vi "Dresden R2R Sputter 03.02.2018 IY24.vi"() -> ()   [LabVIEW 2009] (continued)
                                }
                                frame #4 {
                                n27061 = Wait (ms)(milliseconds to wait=u32 100) -> ()  [unwired: 1 out]
                                n27062 = local write "Parameters_auto_set"(TRUE ("Parameters_auto_set")) -> ()
                                }
                                frame #5 {
                                n27063 = while {
                                i -> [w32211]
                                stop <- w32207 stop-if-true
                                n27064 = Wait Until Next ms Multiple(millisecond multiple=u32 300) -> ()  [unwired: 1 out]
                                n27065 = Greater?(x=w32211, y=100) -> (0:w32208:bool)
                                n27066 = local read "Parameters_auto_set"() -> (w32212:bool)
                                n27067 = case shown="False" w32212 {
                                tunnel: [TRUE FALSE] -> w32209
                                frame #0 {
                                }
                                frame #1 {
                                }
                                }
                                n27068 = Or(x=w32209, y=w32208) -> (x .or. y?=w32207:bool)
                                }
                                }
                                frame #6 {
                                n27069 = local read "R Tension Value"() -> (w32216:dbl)
                                n27070 = Wait (ms)(milliseconds to wait=u32 200) -> ()  [unwired: 1 out]
                                n27071 = local write "TC1_set_value"(w32216) -> ()
                                }
                                frame #7 {
                                n27072 = local write "TC1_auto_set"(TRUE ("TC1_auto_set")) -> ()
                                }
                                frame #8 {
                                w32220 = u16 2 items=["1", "2", "3", "4"] ("Target Chamber Sensor")
                                n27073 = local write "Target Chamber Sensor"(w32220) -> ()
                                n27074 = Wait (ms)(milliseconds to wait=u32 200) -> ()  [unwired: 1 out]
                                }
                                frame #9 {
                                n27075 = local read "Total length"() -> (w32221:dbl)
                                n27076 = local write "Region"(w32221) -> ()
                                }
                                frame #10 {
                                n27077 = local read "Semi"() -> (w32222:bool)
                                n27078 = case shown="False" w32222 {
                                frame #0 {
                                n27079 = stacked-sequence {
                                frame #0 {
                                # "Gas Flow"
                                n27080 = stacked-sequence {
                                frame #0 {
                                n27081 = local read "Semi"() -> (w32223:bool)
                                n27082 = case shown="False" w32223 {
                                frame #0 {
                                n27083 = stacked-sequence {
                                frame #0 {
                                n27084 = local read "Semi"() -> (w32224:bool)
                                n27085 = case shown="False" w32224 {
                                frame #0 {
                                n27086 = local read "R Argon Flow sccm"() -> (w32225:dbl)
                                n27087 = local write "Ar_sccm3_4"(w32225) -> ()
                                }
                                frame #1 {
                                }
                                }
                                }
                                frame #1 {
                                n27088 = local read "Semi"() -> (w32226:bool)
                                n27089 = case shown="False" w32226 {
                                frame #0 {
                                n27090 = local write "Mfc2_Ar _3_4_set"(TRUE ("Mfc_Ar _1_2_set")) -> ()
                                }
                                frame #1 {
                                }
                                }
                                }
                                frame #2 {
                                n27091 = local read "Semi"() -> (w32228:bool)
                                n27092 = case shown="False" w32228 {
                                frame #0 {
                                n27093 = while {
                                i -> [w32231]
                                stop <- w32233 stop-if-true
                                n27094 = Greater?(x=w32231, y=50) -> (0:w32230:bool)
                                n27095 = local read "Semi"() -> (w32229:bool)
                                n27096 = Or(x=w32229, y=w32230) -> (x .or. y?=w32233:bool)
                                }
                                }
                                frame #1 {
                                }
                                }
                                }
                                frame #3 {
                                n27097 = local read "Semi"() -> (w32234:bool)
                                n27098 = case shown="False" w32234 {
                                frame #0 {
                                n27099 = local read "Ar_sccm_act 2"() -> (w32235:dbl)
                                n27100 = Greater?(x=w32235, y=1) -> (0:w32236:bool)
                                n27101 = case shown="False" w32236 {
                                frame #0 {
                                n27102 = local read "R Argon Flow sccm"() -> (w32238:dbl)
                                n27103 = local write "Ar_sccm3_4"(w32238) -> ()
                                }
                                frame #1 {
                                }
                                }
                                }
                                frame #1 {
                                }
                                }
                                }
                                frame #4 {
                                n27104 = local read "Semi"() -> (w32239:bool)
                                n27105 = case shown="False" w32239 {
                                frame #0 {
                                n27106 = local read "Ar_sccm_act 2"() -> (w32240:dbl)
                                n27107 = Greater?(x=w32240, y=1) -> (0:w32241:bool)
                                n27108 = case shown="False" w32241 {
                                frame #0 {
                                n27109 = while {
                                i -> [w32244]
                                stop <- w32248 stop-if-true
                                n27110 = Greater?(x=w32244, y=50) -> (0:w32243:bool)
                                n27111 = local read "Semi"() -> (w32247:bool)
                                n27112 = case shown="False" w32247 {
                                tunnel: [FALSE TRUE] -> w32246
                                frame #0 {
                                n27113 = Wait Until Next ms Multiple(millisecond multiple=u32 200) -> ()  [unwired: 1 out]
                                }
                                frame #1 {
                                }
                                }
                                n27114 = Or(x=w32246, y=w32243) -> (x .or. y?=w32248:bool)
                                }
                                }
                                frame #1 {
                                }
                                }
                                }
                                frame #1 {
                                }
                                }
                                }
                                frame #5 {
                                n27115 = local read "Semi"() -> (w32252:bool)
                                n27116 = case shown="False" w32252 {
                                frame #0 {
                                n27117 = local read "Ar_sccm_act 2"() -> (w32253:dbl)
                                n27118 = Greater?(x=w32253, y=1) -> (0:w32254:bool)
                                n27119 = case shown="False" w32254 {
                                frame #0 {
                                n27120 = local write "Semi"(TRUE ("Semi")) -> ()
                                n27121 = local write "Error Message"("Coating process cancelled.\nPlease check connections." ("Error Message")) -> ()
                                }
                                frame #1 {
                                }
                                }
                                }
                                frame #1 {
                                }
                                }
                                }
                                }
                                }
                                frame #1 {
                                }
                                }
                                }
                                frame #1 {
                                n27122 = local read "Semi"() -> (w32258:bool)
                                n27123 = case shown="False" w32258 {
                                frame #0 {
                                n27124 = local write "SDC1 11"(TRUE ("SDC1 11")) -> ()
                                n27125 = Wait (ms)(milliseconds to wait=u32 1000) -> ()  [unwired: 1 out]
                                }
                                frame #1 {
                                }
                                }
                                }
                                }
                                }
                                frame #1 {
                                # "Set Pressure for ignite plasma"
                                n27126 = stacked-sequence {
                                frame #0 {
                                n27127 = local read "Semi"() -> (w32261:bool)
                                n27128 = case shown="False" w32261 {
                                frame #0 {
                                n27129 = stacked-sequence {
                                frame #0 {
                                n27130 = local read "Semi"() -> (w32262:bool)
                                n27131 = case shown="False" w32262 {
                                frame #0 {
                                n27132 = local write "Set_pressure_value 3"(10.0 ("Set_pressure_value 2")) -> ()
                                }
                                frame #1 {
                                }
                                }
                                }
                                frame #1 {
                                n27133 = local read "Semi"() -> (w32264:bool)
                                n27134 = case shown="False" w32264 {
                                frame #0 {
                                n27135 = Wait (ms)(milliseconds to wait=u32 1000) -> ()  [unwired: 1 out]
                                }
                                frame #1 {
                                }
                                }
                                }
                                frame #2 {
                                n27136 = local read "Semi"() -> (w32266:bool)
                                n27137 = case shown="False" w32266 {
                                frame #0 {
                                n27138 = local write "Pc_bv3_auto_set_pressure"(TRUE ("Pc_bv1_auto_set_pressure")) -> ()
                                }
                                frame #1 {
                                }
                                }
                                }
                                frame #3 {
                                n27139 = local read "Semi"() -> (w32268:bool)
                                n27140 = case shown="False" w32268 {
                                frame #0 {
                                n27141 = while {
                                i -> [w32279]
                                stop <- w32271 stop-if-true
                                w32269 = 10.0 ("Set_pressure_value 2")
                                n27142 = Greater?(x=w32279, y=300) -> (0:w32273:bool)
                                n27143 = Add(x=1.0, y=w32269) -> (x+y=w32275:dbl)
                                n27144 = Subtract(x=w32269, y=1.0) -> (x-y=w32276:dbl)
                                n27145 = local read "Pressure_ch3"() -> (w32270:i32)
                                n27146 = In Range and Coerce(upper limit=w32275, x=w32270, lower limit=w32276) -> (In Range?=w32274:bool)  [unwired: 1 out]
                                n27147 = case shown="False" w32274 {
                                tunnel: [FALSE TRUE] -> w32272
                                frame #0 {
                                n27148 = Wait Until Next ms Multiple(millisecond multiple=u32 200) -> ()  [unwired: 1 out]
                                }
                                frame #1 {
                                }
                                }
                                n27149 = Or(x=w32272, y=w32273) -> (x .or. y?=w32271:bool)
                                }
                                }
                                frame #1 {
                                }
                                }
                                }
                                frame #4 {
                                n27150 = local read "Semi"() -> (w32284:bool)
                                n27151 = case shown="False" w32284 {
                                frame #0 {
                                w32285 = 10.0 ("Set_pressure_value 2")
                                n27152 = Add(x=1.0, y=w32285) -> (x+y=w32288:dbl)
                                n27153 = Subtract(x=w32285, y=1.0) -> (x-y=w32289:dbl)
                                n27154 = local read "Pressure_ch3"() -> (w32286:i32)
                                n27155 = In Range and Coerce(upper limit=w32288, x=w32286, lower limit=w32289) -> (In Range?=w32287:bool)  [unwired: 1 out]
                                n27156 = case shown="False" w32287 {
                                frame #0 {
                                n27157 = local read "R Set Pressure mtorr"() -> (w32292:dbl)
                                n27158 = local write "Set_pressure_value 3"(w32292) -> ()
                                }
                                frame #1 {
                                }
                                }
                                }
                                frame #1 {
                                }
                                }
                                }
                                frame #5 {
                                n27159 = local read "Semi"() -> (w32293:bool)
                                n27160 = case shown="False" w32293 {
                                frame #0 {
                                w32294 = 10.0 ("Set_pressure_value 2")
                                n27161 = Add(x=1.0, y=w32294) -> (x+y=w32297:dbl)
                                n27162 = Subtract(x=w32294, y=1.0) -> (x-y=w32298:dbl)
                                n27163 = local read "Pressure_ch3"() -> (w32295:i32)
                                n27164 = In Range and Coerce(upper limit=w32297, x=w32295, lower limit=w32298) -> (In Range?=w32296:bool)  [unwired: 1 out]
                                n27165 = case shown="False" w32296 {
                                frame #0 {
                                n27166 = local write "Pc_bv3_auto_set_pressure"(TRUE ("Pc_bv1_auto_set_pressure")) -> ()
                                }
                                frame #1 {
                                }
                                }
                                }
                                frame #1 {
                                }
                                }
                                }
                                frame #6 {
                                n27167 = local read "Semi"() -> (w32302:bool)
                                n27168 = case shown="False" w32302 {
                                frame #0 {
                                n27169 = while {
                                i -> [w32313]
                                stop <- w32305 stop-if-true
                                w32303 = 10.0 ("Set_pressure_value 2")
                                n27170 = Greater?(x=w32313, y=300) -> (0:w32307:bool)
                                n27171 = Add(x=1.0, y=w32303) -> (x+y=w32309:dbl)
                                n27172 = Subtract(x=w32303, y=1.0) -> (x-y=w32310:dbl)
                                n27173 = local read "Pressure_ch3"() -> (w32304:i32)
                                n27174 = In Range and Coerce(upper limit=w32309, x=w32304, lower limit=w32310) -> (In Range?=w32308:bool)  [unwired: 1 out]
                                n27175 = case shown="False" w32308 {
                                tunnel: [FALSE TRUE] -> w32306
                                frame #0 {
                                n27176 = Wait Until Next ms Multiple(millisecond multiple=u32 200) -> ()  [unwired: 1 out]
                                }
                                frame #1 {
                                }
                                }
                                n27177 = Or(x=w32306, y=w32307) -> (x .or. y?=w32305:bool)
                                }
                                }
                                frame #1 {
                                }
                                }
                                }
                                frame #7 {
                                n27178 = local read "Semi"() -> (w32318:bool)
                                n27179 = case shown="False" w32318 {
                                frame #0 {
                                n27180 = local read "Set_pressure_value 3"() -> (w32321:dbl)
                                n27181 = Add(x=1.0, y=w32321) -> (x+y=w32322:dbl)
                                n27182 = Subtract(x=w32321, y=1.0) -> (x-y=w32323:dbl)
                                n27183 = local read "Pressure_ch3"() -> (w32319:i32)
                                n27184 = In Range and Coerce(upper limit=w32322, x=w32319, lower limit=w32323) -> (In Range?=w32320:bool)  [unwired: 1 out]
                                n27185 = case shown="False" w32320 {
                                frame #0 {
                                n27186 = local write "Semi"(TRUE ("Semi")) -> ()
                                n27187 = local write "Error Message"("Coating Pressure could not be adjusted !" ("Error Message")) -> ()
                                }
                                frame #1 {
                                }
                                }
                                }
                                frame #1 {
                                }
                                }
                                }
                                }
                                }
                                frame #1 {
                                }
                                }
                                }
                                frame #1 {
                                n27188 = local read "Semi"() -> (w32328:bool)
                                n27189 = case shown="False" w32328 {
                                frame #0 {
                                n27190 = local write "SDC1 9"(TRUE ("SDC1 9")) -> ()
                                n27191 = Wait (ms)(milliseconds to wait=u32 1000) -> ()  [unwired: 1 out]
                                }
                                frame #1 {
                                }
                                }
                                }
                                }
                                }
                                frame #2 {
                                # "Plasma ignite and check"
                                n27192 = stacked-sequence {
                                frame #0 {
                                n27193 = local read "Semi"() -> (w32331:bool)
                                n27194 = case shown="False" w32331 {
                                frame #0 {
                                n27195 = local write "Dc_auto_on"(TRUE ("Dc_auto_on")) -> ()
                                }
                                frame #1 {
                                }
                                }
                                }
                                frame #1 {
                                n27196 = local read "Semi"() -> (w32333:bool)
                                n27197 = case shown="False" w32333 {
                                frame #0 {
                                n27198 = while {
                                i -> [w32343]
                                stop <- w32334 stop-if-true
                                n27199 = Greater Or Equal?(x=w32343, y=240) -> (x >= y?=w32342:bool)
                                n27200 = case shown="True" w32342 {
                                frame #0 {
                                }
                                frame #1 {
                                n27201 = local write "Semi"(TRUE ("Semi")) -> ()
                                }
                                }
                                n27202 = local read "Set DC Power       : 2"() -> (w32339:dbl)
                                n27203 = local read "Actual DC Power : 2"() -> (w32338:dbl)
                                n27204 = Subtract(x=w32339, y=w32338) -> (x-y=w32341:dbl)
                                n27205 = Less?(x=w32341, y=10.0) -> (x < y?=w32336:bool)
                                n27206 = local read "Semi"() -> (w32335:bool)
                                n27207 = Or(x=w32336, y=w32335) -> (x .or. y?=w32334:bool)
                                n27208 = Wait Until Next ms Multiple(millisecond multiple=u32 500) -> ()  [unwired: 1 out]
                                }
                                }
                                frame #1 {
                                }
                                }
                                }
                                }
                                }
                                frame #3 {
                                # "Set Pressure for coating"
                                n27209 = stacked-sequence {
                                frame #0 {
                                n27210 = local read "Semi"() -> (w32346:bool)
                                n27211 = case shown="False" w32346 {
                                frame #0 {
                                n27212 = stacked-sequence {
                                frame #0 {
                                n27213 = local read "Semi"() -> (w32347:bool)
                                n27214 = case shown="False" w32347 {
                                frame #0 {
                                n27215 = local read "R Set Pressure mtorr"() -> (w32348:dbl)
                                n27216 = local write "Set_pressure_value 3"(w32348) -> ()
                                }
                                frame #1 {
                                }
                                }
                                }
                                frame #1 {
                                n27217 = local read "Semi"() -> (w32349:bool)
                                n27218 = case shown="False" w32349 {
                                frame #0 {
                                n27219 = Wait (ms)(milliseconds to wait=u32 200) -> ()  [unwired: 1 out]
                                }
                                frame #1 {
                                }
                                }
                                }
                                frame #2 {
                                n27220 = local read "Semi"() -> (w32351:bool)
                                n27221 = case shown="False" w32351 {
                                frame #0 {
                                n27222 = local write "Pc_bv3_auto_set_pressure"(TRUE ("Pc_bv1_auto_set_pressure")) -> ()
                                }
                                frame #1 {
                                }
                                }
                                }
                                frame #3 {
                                n27223 = local read "Semi"() -> (w32353:bool)
                                n27224 = case shown="False" w32353 {
                                frame #0 {
                                n27225 = while {
                                i -> [w32364]
                                stop <- w32356 stop-if-true
                                n27226 = local read "Set_pressure_value 3"() -> (w32354:dbl)
                                n27227 = Greater?(x=w32364, y=300) -> (0:w32358:bool)
                                n27228 = Add(x=1.0, y=w32354) -> (x+y=w32360:dbl)
                                n27229 = Subtract(x=w32354, y=1.0) -> (x-y=w32361:dbl)
                                n27230 = local read "Pressure_ch3"() -> (w32355:i32)
                                n27231 = In Range and Coerce(upper limit=w32360, x=w32355, lower limit=w32361) -> (In Range?=w32359:bool)  [unwired: 1 out]
                                n27232 = case shown="False" w32359 {
                                tunnel: [FALSE TRUE] -> w32357
                                frame #0 {
                                n27233 = Wait Until Next ms Multiple(millisecond multiple=u32 200) -> ()  [unwired: 1 out]
                                }
                                frame #1 {
                                }
                                }
                                n27234 = Or(x=w32357, y=w32358) -> (x .or. y?=w32356:bool)
                                }
                                }
                                frame #1 {
                                }
                                }
                                }
                                frame #4 {
                                n27235 = local read "Semi"() -> (w32369:bool)
                                n27236 = case shown="False" w32369 {
                                frame #0 {
                                n27237 = local read "Set_pressure_value 3"() -> (w32370:dbl)
                                n27238 = Add(x=1.0, y=w32370) -> (x+y=w32373:dbl)
                                n27239 = Subtract(x=w32370, y=1.0) -> (x-y=w32374:dbl)
                                n27240 = local read "Pressure_ch3"() -> (w32371:i32)
                                n27241 = In Range and Coerce(upper limit=w32373, x=w32371, lower limit=w32374) -> (In Range?=w32372:bool)  [unwired: 1 out]
                                n27242 = case shown="False" w32372 {
                                frame #0 {
                                n27243 = local read "R Set Pressure mtorr"() -> (w32377:dbl)
                                n27244 = local write "Set_pressure_value 3"(w32377) -> ()
                                }
                                frame #1 {
                                }
                                }
                                }
                                frame #1 {
                                }
                                }
                                }
                                frame #5 {
                                n27245 = local read "Semi"() -> (w32378:bool)
                                n27246 = case shown="False" w32378 {
                                frame #0 {
                                n27247 = local read "Set_pressure_value 3"() -> (w32379:dbl)
                                n27248 = Add(x=1.0, y=w32379) -> (x+y=w32382:dbl)
                                n27249 = Subtract(x=w32379, y=1.0) -> (x-y=w32383:dbl)
                                n27250 = local read "Pressure_ch3"() -> (w32380:i32)
                                n27251 = In Range and Coerce(upper limit=w32382, x=w32380, lower limit=w32383) -> (In Range?=w32381:bool)  [unwired: 1 out]
                                n27252 = case shown="False" w32381 {
                                frame #0 {
                                n27253 = local write "Pc_bv3_auto_set_pressure"(TRUE ("Pc_bv1_auto_set_pressure")) -> ()
                                }
                                frame #1 {
                                }
                                }
                                }
                                frame #1 {
                                }
                                }
                                }
                                frame #6 {
                                n27254 = local read "Semi"() -> (w32387:bool)
                                n27255 = case shown="False" w32387 {
                                frame #0 {
                                n27256 = while {
                                i -> [w32398]
                                stop <- w32389 stop-if-true
                                n27257 = local read "Set_pressure_value 3"() -> (w32393:dbl)
                                n27258 = Greater?(x=w32398, y=300) -> (0:w32391:bool)
                                n27259 = Add(x=1.0, y=w32393) -> (x+y=w32394:dbl)
                                n27260 = Subtract(x=w32393, y=1.0) -> (x-y=w32395:dbl)
                                n27261 = local read "Pressure_ch3"() -> (w32388:i32)
                                n27262 = In Range and Coerce(upper limit=w32394, x=w32388, lower limit=w32395) -> (In Range?=w32392:bool)  [unwired: 1 out]
                                n27263 = case shown="False" w32392 {
                                tunnel: [FALSE TRUE] -> w32390
                                frame #0 {
                                n27264 = Wait Until Next ms Multiple(millisecond multiple=u32 200) -> ()  [unwired: 1 out]
                                }
                                frame #1 {
                                }
                                }
                                n27265 = Or(x=w32390, y=w32391) -> (x .or. y?=w32389:bool)
                                }
                                }
                                frame #1 {
                                }
                                }
                                }
                                frame #7 {
                                n27266 = local read "Semi"() -> (w32403:bool)
                                n27267 = case shown="False" w32403 {
                                frame #0 {
                                n27268 = local read "Set_pressure_value 3"() -> (w32406:dbl)
                                n27269 = Add(x=1.0, y=w32406) -> (x+y=w32407:dbl)
                                n27270 = Subtract(x=w32406, y=1.0) -> (x-y=w32408:dbl)
                                n27271 = local read "Pressure_ch3"() -> (w32404:i32)
                                n27272 = In Range and Coerce(upper limit=w32407, x=w32404, lower limit=w32408) -> (In Range?=w32405:bool)  [unwired: 1 out]
                                n27273 = case shown="False" w32405 {
                                frame #0 {
                                n27274 = local write "Semi"(TRUE ("Semi")) -> ()
                                n27275 = local write "Error Message"("Coating Pressure could not be adjusted !" ("Error Message")) -> ()
                                }
                                frame #1 {
                                }
                                }
                                }
                                frame #1 {
                                }
                                }
                                }
                                }
                                }
                                frame #1 {
                                }
                                }
                                }
                                frame #1 {
                                n27276 = local read "Semi"() -> (w32413:bool)
                                n27277 = case shown="False" w32413 {
                                frame #0 {
                                n27278 = local write "SDC1 9"(TRUE ("SDC1 9")) -> ()
                                n27279 = Wait (ms)(milliseconds to wait=u32 1000) -> ()  [unwired: 1 out]
                                }
                                frame #1 {
                                }
                                }
                                }
                                }
                                }
                                }
                                }
                                frame #1 {
                                }
                                }
                                }
                                frame #11 {
                                n27280 = local read "Semi"() -> (w32416:bool)
                                n27281 = case shown="False" w32416 {
                                frame #0 {
                                n27282 = local write "Start_roll"(TRUE ("Start_roll")) -> ()
                                n27283 = Wait (ms)(milliseconds to wait=u32 300) -> ()  [unwired: 1 out]
                                }
                                frame #1 {
                                }
                                }
                                }
                                frame #12 {
                                n27284 = local read "Semi"() -> (w32419:bool)
                                n27285 = case shown="False" w32419 {
                                frame #0 {
                                n27286 = stacked-sequence {
                                frame #0 {
                                n27287 = local read "R Single DC Step1 Coating Power Active"() -> (w32420:bool)
                                n27288 = case shown="True" w32420 {
                                frame #0 {
                                }
                                frame #1 {
                                n27289 = while {
                                stop <- w32422 stop-if-true
                                n27290 = local read "R Single DC Interval length"() -> (w32426:dbl)
                                n27291 = local read "Actual Length"() -> (w32425:dbl)
                                n27292 = Greater Or Equal?(x=w32425, y=w32426) -> (x >= y?=w32424:bool)
                                n27293 = local read "Semi"() -> (w32423:bool)
                                n27294 = Or(x=w32424, y=w32423) -> (x .or. y?=w32422:bool)
                                n27295 = Wait Until Next ms Multiple(millisecond multiple=u32 300) -> ()  [unwired: 1 out]
                                }
                                }
                                }
                                }
                                frame #1 {
                                n27296 = local read "R Single DC Step2 Coating Power Active"() -> (w32427:bool)
                                n27297 = case shown="True" w32427 {
                                frame #0 {
                                }
                                frame #1 {
                                n27298 = stacked-sequence {
                                frame #0 {
                                n27299 = local read "Semi"() -> (w32428:bool)
                                n27300 = case shown="False" w32428 {
                                frame #0 {
                                n27301 = local read "R Single DC Step2 Coating Power"() -> (w32430:dbl)
                                n27302 = Wait (ms)(milliseconds to wait=u32 200) -> ()  [unwired: 1 out]
                                n27303 = local write "Set DC Power       : 2"(w32430) -> ()
                                }
                                frame #1 {
                                }
                                }
                                }
                                frame #1 {
                                n27304 = local read "Semi"() -> (w32431:bool)
                                n27305 = case shown="False" w32431 {
                                frame #0 {
                                n27306 = local write "Dc_auto_set"(TRUE ("Dc_auto_set")) -> ()
                                }
                                frame #1 {
                                }
                                }
                                }
                                frame #2 {
                                n27307 = while {
                                stop <- w32437 stop-if-true
                                n27308 = local read "R Single DC Interval length"() -> (w32436:dbl)
                                n27309 = local read "Actual Length"() -> (w32440:dbl)
                                n27310 = Multiply(x=w32436, y=2.0) -> (x*y=w32434:dbl)
                                n27311 = Greater Or Equal?(x=w32440, y=w32434) -> (x >= y?=w32439:bool)
                                n27312 = local read "Semi"() -> (w32438:bool)
                                n27313 = Or(x=w32439, y=w32438) -> (x .or. y?=w32437:bool)
                                n27314 = Wait Until Next ms Multiple(millisecond multiple=u32 300) -> ()  [unwired: 1 out]
                                }
                                }
                                }
                                }
                                }
                                }
                                frame #2 {
                                n27315 = local read "R Single DC Step3 Coating Power Active"() -> (w32441:bool)
                                n27316 = case shown="True" w32441 {
                                frame #0 {
                                }
                                frame #1 {
                                n27317 = stacked-sequence {
                                frame #0 {
                                n27318 = local read "Semi"() -> (w32442:bool)
                                n27319 = case shown="False" w32442 {
                                frame #0 {
                                n27320 = local read "R Single DC Step3 Coating Power"() -> (w32444:dbl)
                                n27321 = Wait (ms)(milliseconds to wait=u32 200) -> ()  [unwired: 1 out]
                                n27322 = local write "Set DC Power       : 2"(w32444) -> ()
                                }
                                frame #1 {
                                }
                                }
                                }
                                frame #1 {
                                n27323 = local read "Semi"() -> (w32445:bool)
                                n27324 = case shown="False" w32445 {
                                frame #0 {
                                n27325 = local write "Dc_auto_set"(TRUE ("Dc_auto_set")) -> ()
                                }
                                frame #1 {
                                }
                                }
                                }
                                frame #2 {
                                n27326 = while {
                                stop <- w32451 stop-if-true
                                n27327 = local read "R Single DC Interval length"() -> (w32450:dbl)
                                n27328 = local read "Actual Length"() -> (w32454:dbl)
                                n27329 = Multiply(x=w32450, y=3.0) -> (x*y=w32448:dbl)
                                n27330 = Greater Or Equal?(x=w32454, y=w32448) -> (x >= y?=w32453:bool)
                                n27331 = local read "Semi"() -> (w32452:bool)
                                n27332 = Or(x=w32453, y=w32452) -> (x .or. y?=w32451:bool)
                                n27333 = Wait Until Next ms Multiple(millisecond multiple=u32 300) -> ()  [unwired: 1 out]
                                }
                                }
                                }
                                }
                                }
                                }
                                frame #3 {
                                n27334 = local read "R Single DC Step4 Coating Power Active"() -> (w32455:bool)
                                n27335 = case shown="True" w32455 {
                                frame #0 {
                                }
                                frame #1 {
                                n27336 = stacked-sequence {
                                frame #0 {
                                n27337 = local read "Semi"() -> (w32456:bool)
                                n27338 = case shown="False" w32456 {
                                frame #0 {
                                n27339 = local read "R Single DC Step4 Coating Power"() -> (w32458:dbl)
                                n27340 = Wait (ms)(milliseconds to wait=u32 200) -> ()  [unwired: 1 out]
                                n27341 = local write "Set DC Power       : 2"(w32458) -> ()
                                }
                                frame #1 {
                                }
                                }
                                }
                                frame #1 {
                                n27342 = local read "Semi"() -> (w32459:bool)
                                n27343 = case shown="False" w32459 {
                                frame #0 {
                                n27344 = local write "Dc_auto_set"(TRUE ("Dc_auto_set")) -> ()
                                }
                                frame #1 {
                                }
                                }
                                }
                                frame #2 {
                                n27345 = while {
                                stop <- w32465 stop-if-true
                                n27346 = local read "R Single DC Interval length"() -> (w32464:dbl)
                                n27347 = local read "Actual Length"() -> (w32468:dbl)
                                n27348 = Multiply(x=w32464, y=4.0) -> (x*y=w32462:dbl)
                                n27349 = Greater Or Equal?(x=w32468, y=w32462) -> (x >= y?=w32467:bool)
                                n27350 = local read "Semi"() -> (w32466:bool)
                                n27351 = Or(x=w32467, y=w32466) -> (x .or. y?=w32465:bool)
                                n27352 = Wait Until Next ms Multiple(millisecond multiple=u32 300) -> ()  [unwired: 1 out]
                                }
                                }
                                }
                                }
                                }
                                }
                                frame #4 {
                                n27353 = local read "R Single DC Step5 Coating Power Active"() -> (w32469:bool)
                                n27354 = case shown="True" w32469 {
                                frame #0 {
                                }
                                frame #1 {
                                n27355 = stacked-sequence {
                                frame #0 {
                                n27356 = local read "Semi"() -> (w32470:bool)
                                n27357 = case shown="False" w32470 {
                                frame #0 {
                                n27358 = local read "R Single DC Step5 Coating Power"() -> (w32472:dbl)
                                n27359 = Wait (ms)(milliseconds to wait=u32 200) -> ()  [unwired: 1 out]
                                n27360 = local write "Set DC Power       : 2"(w32472) -> ()
                                }
                                frame #1 {
                                }
                                }
                                }
                                frame #1 {
                                n27361 = local read "Semi"() -> (w32473:bool)
                                n27362 = case shown="False" w32473 {
                                frame #0 {
                                n27363 = local write "Dc_auto_set"(TRUE ("Dc_auto_set")) -> ()
                                }
                                frame #1 {
                                }
                                }
                                }
                                frame #2 {
                                n27364 = while {
                                stop <- w32479 stop-if-true